vi "Dresden R2R Sputter 03.02.2018 IY24.vi"() -> ()   [LabVIEW 2009] (continued)
        n9883 = Build Array(i32? 49407 ("element")) -> (w15888)
        n9884 = call <vilib>:"MB Serial Master Query Write Multiple Registers (poly).vi"(0:w15891, 1:i16? 320 ("Starting Address"), 2:w15888, 5:w15892, 6:w15880) -> (14:w15882, 19:w15881)  [unwired: 12 in, 1 out]
      }
      frame #9 {
        w15902 = data[3B] ("Serial Parameters")
        n9885 = Type Cast(type=data[3B], x="TC2_overspeed_value") -> (*(type *) &x=w15894)
        n9886 = Build Array(w15894) -> (w15895)
        n9887 = Increment(x=i16? 130) -> (x+1=w15899)
        n9888 = call <vilib>:"MB Serial Master Query Write Multiple Registers (poly).vi"(0:w15901, 1:w15899, 2:w15895, 5:w15900, 6:w15902) -> (14:w15909, 19:w15908)  [unwired: 12 in, 1 out]
        n9889 = local write "TC2_overspeed_set"(i16? 0 ("TC2_overspeed_set")) -> ()
        n9890 = Build Array(i32? 49152 ("element")) -> (w15907)
        n9891 = call <vilib>:"MB Serial Master Query Write Multiple Registers (poly).vi"(0:w15909, 1:i16? 320 ("Starting Address"), 2:w15907, 5:w15908, 6:w15902) -> (14:w15913, 19:w15914)  [unwired: 12 in, 1 out]
        n9892 = Build Array(i32? 49407 ("element")) -> (w15910)
        n9893 = call <vilib>:"MB Serial Master Query Write Multiple Registers (poly).vi"(0:w15913, 1:i16? 320 ("Starting Address"), 2:w15910, 5:w15914, 6:w15902) -> (14:w15904, 19:w15903)  [unwired: 12 in, 1 out]
      }
      frame #10 {
        w15924 = data[3B] ("Serial Parameters")
        n9894 = Type Cast(type=data[3B], x="TC2_AO1_upper_limit_value") -> (*(type *) &x=w15916)
        n9895 = Build Array(w15916) -> (w15917)
        n9896 = Increment(x=i16? 168) -> (x+1=w15921)
        n9897 = call <vilib>:"MB Serial Master Query Write Multiple Registers (poly).vi"(0:w15923, 1:w15921, 2:w15917, 5:w15922, 6:w15924) -> (14:w15931, 19:w15930)  [unwired: 12 in, 1 out]
        n9898 = local write "TC2_AO1_upper_limit_set"(i16? 0 ("TC2_AO1_upper_limit_set")) -> ()
        n9899 = Build Array(i32? 49152 ("element")) -> (w15929)
        n9900 = call <vilib>:"MB Serial Master Query Write Multiple Registers (poly).vi"(0:w15931, 1:i16? 320 ("Starting Address"), 2:w15929, 5:w15930, 6:w15924) -> (14:w15935, 19:w15936)  [unwired: 12 in, 1 out]
        n9901 = Build Array(i32? 49407 ("element")) -> (w15932)
        n9902 = call <vilib>:"MB Serial Master Query Write Multiple Registers (poly).vi"(0:w15935, 1:i16? 320 ("Starting Address"), 2:w15932, 5:w15936, 6:w15924) -> (14:w15926, 19:w15925)  [unwired: 12 in, 1 out]
      }
      frame #11 {
        w15946 = data[3B] ("Serial Parameters")
        n9903 = Type Cast(type=data[3B], x="TC2_AO1_bottom_limit_value") -> (*(type *) &x=w15938)
        n9904 = Build Array(w15938) -> (w15939)
        n9905 = Increment(x=i16? 166) -> (x+1=w15943)
        n9906 = local write "TC2_AO1_bottom_limit_set"(i16? 0 ("TC2_AO1_bottom_limit_set")) -> ()
        n9907 = call <vilib>:"MB Serial Master Query Write Multiple Registers (poly).vi"(0:w15945, 1:w15943, 2:w15939, 5:w15944, 6:w15946) -> (14:w15953, 19:w15952)  [unwired: 12 in, 1 out]
        n9908 = Build Array(i32? 49152 ("element")) -> (w15951)
        n9909 = call <vilib>:"MB Serial Master Query Write Multiple Registers (poly).vi"(0:w15953, 1:i16? 320 ("Starting Address"), 2:w15951, 5:w15952, 6:w15946) -> (14:w15957, 19:w15958)  [unwired: 12 in, 1 out]
        n9910 = Build Array(i32? 49407 ("element")) -> (w15954)
        n9911 = call <vilib>:"MB Serial Master Query Write Multiple Registers (poly).vi"(0:w15957, 1:i16? 320 ("Starting Address"), 2:w15954, 5:w15958, 6:w15946) -> (14:w15948, 19:w15947)  [unwired: 12 in, 1 out]
      }
      frame #12 {
        w15968 = data[3B] ("Serial Parameters")
        n9912 = Type Cast(type=data[3B], x=data[5B] ("TC1_AO1_bottom_limit_value 2")) -> (*(type *) &x=w15960)
        n9913 = Build Array(w15960) -> (w15961)
        n9914 = Increment(x=i16? 198) -> (x+1=w15965)
        n9915 = local write "TC2_AO1_polarity(neg_to_pos)"(i16? 0 ("TC2_AO1_polarity(neg_to_pos)")) -> ()
        n9916 = call <vilib>:"MB Serial Master Query Write Multiple Registers (poly).vi"(0:w15967, 1:w15965, 2:w15961, 5:w15966, 6:w15968) -> (14:w15975, 19:w15974)  [unwired: 12 in, 1 out]
        n9917 = Build Array(i32? 49152 ("element")) -> (w15973)
        n9918 = call <vilib>:"MB Serial Master Query Write Multiple Registers (poly).vi"(0:w15975, 1:i16? 320 ("Starting Address"), 2:w15973, 5:w15974, 6:w15968) -> (14:w15979, 19:w15980)  [unwired: 12 in, 1 out]
        n9919 = Build Array(i32? 49407 ("element")) -> (w15976)
        n9920 = call <vilib>:"MB Serial Master Query Write Multiple Registers (poly).vi"(0:w15979, 1:i16? 320 ("Starting Address"), 2:w15976, 5:w15980, 6:w15968) -> (14:w15970, 19:w15969)  [unwired: 12 in, 1 out]
      }
      frame #13 {
        w15990 = data[3B] ("Serial Parameters")
        n9921 = Type Cast(type=data[3B], x=sgl? 1 ("TC1_AO1_bottom_limit_value 2")) -> (*(type *) &x=w15982)
        n9922 = Build Array(w15982) -> (w15983)
        n9923 = Increment(x=i16? 198) -> (x+1=w15987)
        n9924 = local write "TC2_AO1_polarity(pos_to_neg)"(i16? 0 ("TC2_AO1_polarity(pos_to_neg)")) -> ()
        n9925 = call <vilib>:"MB Serial Master Query Write Multiple Registers (poly).vi"(0:w15989, 1:w15987, 2:w15983, 5:w15988, 6:w15990) -> (14:w15997, 19:w15996)  [unwired: 12 in, 1 out]
        n9926 = Build Array(i32? 49152 ("element")) -> (w15995)
        n9927 = call <vilib>:"MB Serial Master Query Write Multiple Registers (poly).vi"(0:w15997, 1:i16? 320 ("Starting Address"), 2:w15995, 5:w15996, 6:w15990) -> (14:w16001, 19:w16002)  [unwired: 12 in, 1 out]
        n9928 = Build Array(i32? 49407 ("element")) -> (w15998)
        n9929 = call <vilib>:"MB Serial Master Query Write Multiple Registers (poly).vi"(0:w16001, 1:i16? 320 ("Starting Address"), 2:w15998, 5:w16002, 6:w15990) -> (14:w15992, 19:w15991)  [unwired: 12 in, 1 out]
      }
      frame #14 {
        w16012 = data[3B] ("Serial Parameters")
        n9930 = Type Cast(type=data[3B], x=sgl? 2 ("TC1_AO1_bottom_limit_value 2")) -> (*(type *) &x=w16004)
        n9931 = local write "TC2_display_tension_set"(i16? 0 ("TC2_display_tension")) -> ()
        n9932 = Build Array(w16004) -> (w16005)
        n9933 = Increment(x=i16? 8) -> (x+1=w16009)
        n9934 = call <vilib>:"MB Serial Master Query Write Multiple Registers (poly).vi"(0:w16011, 1:w16009, 2:w16005, 5:w16010, 6:w16012) -> (14:w16019, 19:w16018)  [unwired: 12 in, 1 out]
        n9935 = Build Array(i32? 49152 ("element")) -> (w16017)
        n9936 = call <vilib>:"MB Serial Master Query Write Multiple Registers (poly).vi"(0:w16019, 1:i16? 320 ("Starting Address"), 2:w16017, 5:w16018, 6:w16012) -> (14:w16023, 19:w16024)  [unwired: 12 in, 1 out]
        n9937 = Build Array(i32? 49407 ("element")) -> (w16020)
        n9938 = call <vilib>:"MB Serial Master Query Write Multiple Registers (poly).vi"(0:w16023, 1:i16? 320 ("Starting Address"), 2:w16020, 5:w16024, 6:w16012) -> (14:w16014, 19:w16013)  [unwired: 12 in, 1 out]
      }
      frame #15 {
        w16034 = data[3B] ("Serial Parameters")
        n9939 = Type Cast(type=data[3B], x=sgl? 5 ("TC1_AO1_bottom_limit_value 2")) -> (*(type *) &x=w16026)
        n9940 = Build Array(w16026) -> (w16027)
        n9941 = Increment(x=i16? 8) -> (x+1=w16031)
        n9942 = call <vilib>:"MB Serial Master Query Write Multiple Registers (poly).vi"(0:w16033, 1:w16031, 2:w16027, 5:w16032, 6:w16034) -> (14:w16041, 19:w16040)  [unwired: 12 in, 1 out]
        n9943 = local write "TC2_display_AO1_set"(i16? 0 ("TC2_display_tension")) -> ()
        n9944 = Build Array(i32? 49152 ("element")) -> (w16039)
        n9945 = call <vilib>:"MB Serial Master Query Write Multiple Registers (poly).vi"(0:w16041, 1:i16? 320 ("Starting Address"), 2:w16039, 5:w16040, 6:w16034) -> (14:w16045, 19:w16046)  [unwired: 12 in, 1 out]
        n9946 = Build Array(i32? 49407 ("element")) -> (w16042)
        n9947 = call <vilib>:"MB Serial Master Query Write Multiple Registers (poly).vi"(0:w16045, 1:i16? 320 ("Starting Address"), 2:w16042, 5:w16046, 6:w16034) -> (14:w16036, 19:w16035)  [unwired: 12 in, 1 out]
      }
      frame #16 {
        w16056 = data[3B] ("Serial Parameters")
        n9948 = Type Cast(type=data[3B], x=sgl? 4 ("TC1_AO1_bottom_limit_value 2")) -> (*(type *) &x=w16048)
        n9949 = local write "TC2_display_tension_actual"(i16? 0 ("TC2_display_tension")) -> ()
        n9950 = Build Array(w16048) -> (w16049)
        n9951 = Increment(x=i16? 10) -> (x+1=w16053)
        n9952 = call <vilib>:"MB Serial Master Query Write Multiple Registers (poly).vi"(0:w16055, 1:w16053, 2:w16049, 5:w16054, 6:w16056) -> (14:w16063, 19:w16062)  [unwired: 12 in, 1 out]
        n9953 = Build Array(i32? 49152 ("element")) -> (w16061)
        n9954 = call <vilib>:"MB Serial Master Query Write Multiple Registers (poly).vi"(0:w16063, 1:i16? 320 ("Starting Address"), 2:w16061, 5:w16062, 6:w16056) -> (14:w16067, 19:w16068)  [unwired: 12 in, 1 out]
        n9955 = Build Array(i32? 49407 ("element")) -> (w16064)
        n9956 = call <vilib>:"MB Serial Master Query Write Multiple Registers (poly).vi"(0:w16067, 1:i16? 320 ("Starting Address"), 2:w16064, 5:w16068, 6:w16056) -> (14:w16058, 19:w16057)  [unwired: 12 in, 1 out]
      }
      frame #17 {
        w16078 = data[3B] ("Serial Parameters")
        n9957 = Type Cast(type=data[3B], x=data[5B] ("TC1_AO1_bottom_limit_value 2")) -> (*(type *) &x=w16070)
        n9958 = Build Array(w16070) -> (w16071)
        n9959 = Increment(x=i16? 10) -> (x+1=w16075)
        n9960 = call <vilib>:"MB Serial Master Query Write Multiple Registers (poly).vi"(0:w16077, 1:w16075, 2:w16071, 5:w16076, 6:w16078) -> (14:w16085, 19:w16084)  [unwired: 12 in, 1 out]
        n9961 = local write "TC2_display_AO1_actual"(i16? 0 ("TC2_display_tension")) -> ()
        n9962 = Build Array(i32? 49152 ("element")) -> (w16083)
        n9963 = call <vilib>:"MB Serial Master Query Write Multiple Registers (poly).vi"(0:w16085, 1:i16? 320 ("Starting Address"), 2:w16083, 5:w16084, 6:w16078) -> (14:w16089, 19:w16090)  [unwired: 12 in, 1 out]
        n9964 = Build Array(i32? 49407 ("element")) -> (w16086)
        n9965 = call <vilib>:"MB Serial Master Query Write Multiple Registers (poly).vi"(0:w16089, 1:i16? 320 ("Starting Address"), 2:w16086, 5:w16090, 6:w16078) -> (14:w16080, 19:w16079)  [unwired: 12 in, 1 out]
      }
      frame #18 {
        n9966 = Build Array(i16? 21767) -> (w16097)
        n9967 = call <vilib>:"MB Serial Master Query Write Multiple Registers (poly).vi"(0:w16099, 1:i16? 322 ("x"), 2:w16097, 5:w16098, 6:data[3B] ("Serial Parameters")) -> (14:w16092, 19:w16093)  [unwired: 12 in, 1 out]
        n9968 = local write "TC2_tare_function"(i16? 0 ("TC2_tare_function")) -> ()
        n9969 = Build Array(i32? 49407 ("element")) -> (w16102)
        n9970 = call <vilib>:"MB Serial Master Query Write Multiple Registers (poly).vi"(0:w16092, 1:i16? 320 ("Starting Address"), 2:w16102, 5:w16093) -> (14:w16101, 19:w16100)  [unwired: 13 in, 1 out]
      }
    }
  }
  n9971 = while {
    tunnel: [w16539] -> w773
    tunnel: [w16538] -> w745
    tunnel: w772 -> [w16537]
    tunnel: w746 -> [w16536]
    tunnel: "milliseconds to wait 3" -> [w16534]
    stop <- FALSE stop-if-true
    n9972 = stacked-sequence {
      tunnel: [w16544 _] -> w16539
      tunnel: [w16543 _] -> w16538
      tunnel: w16537 -> [w16542 _]
      tunnel: w16536 -> [w16541 _]
      tunnel: w16534 -> [w16540 _]
      frame #0 {
        n9973 = stacked-sequence {
          tunnel: w16541 -> [w16563 _ _ _ _ _ _ _ _ _]
          tunnel: w16542 -> [w16562 _ _ _ _ _ _ _ _ _]
          tunnel: [_ _ _ _ _ _ _ _ w16901 _] -> w16543
          tunnel: [_ _ _ _ _ _ _ _ w16900 _] -> w16544
          tunnel: w16540 -> [_ w16637 _ w16656 _ w16711 _ w16887 _ w16920]
          frame #0 {
            # "Digital I/O & Analog \nOutput Part"
            n9974 = call-poly <vilib>:"MB Serial Master Query (poly).vi"("VISA resource name"=w16563, "Starting Address"=u16 0, "Quantity"=u16 8, "error in"=w16562, "Serial Parameters"=T39 {"Mode"=enum."RTU", "Slave Address"=1}) -> ("VISA resource name out"=w16560:refnum<visa-resource-name>, "Discrete Inputs"=w16590:bool[], "error out"=w16561:errorcluster)  [unwired: 1 in, 11 out]
            n9975 = Index Array(array=w16590, index=5) -> (element=w16553:bool)
            "Ch2_Pl_vbv_di" <- w16553
            n9976 = Index Array(array=w16590, index=6) -> (element=w16585:bool)
            "Ch2_Pl_atm_di" <- w16585
            n9977 = Index Array(array=w16590, index=0) -> (element=w16588:bool)
            "Ch2_Mp_di" <- w16588
            n9978 = Index Array(array=w16590, index=1) -> (element=w16587:bool)
            "Ch2_Tp_bv_di" <- w16587
            n9979 = Index Array(array=w16590, index=2) -> (element=w16550:bool)
            "Ch2_Bg_bv_di" <- w16550
            n9980 = Index Array(array=w16590, index=3) -> (element=w16586:bool)
            "Ch2_Ch_vbv_di" <- w16586
            n9981 = Index Array(array=w16590, index=4) -> (element=w16549:bool)
            "Ch2_Ch_atm_di" <- w16549
            n9982 = Index Array(array=w16590, index=7) -> (element=w16548:bool)
            "Ch2_Cc_on_off_di" <- w16548
            n9983 = local write "Ch2_Ch_vbv_on"(w16586) -> ()
            n9984 = local write "Ch2_Ch_atm_on"(w16549) -> ()
            n9985 = local write "Ch2_Bg_bv_on"(w16550) -> ()
            n9986 = local write "ch2_bg_bv_on_top"(w16550) -> ()
            n9987 = local write "ch2_cc_on_top"(w16548) -> ()
            n9988 = local write "Ch2_Tp_bv_on"(w16587) -> ()
            n9989 = local write "Ch2_Pl_atm_on"(w16585) -> ()
            n9990 = local write "Ch2_Ch_cc_on"(w16548) -> ()
            n9991 = local write "Ch2_Mp_on"(w16588) -> ()
            n9992 = local write "Ch2_Pl_vbv_on"(w16553) -> ()
            n9993 = local write "ch2_atm_on_top"(w16549) -> ()
            n9994 = local read "Load_dido"() -> (w16552:bool)
            n9995 = call-poly <vilib>:"MB Serial Master Query (poly).vi"("VISA resource name"=w16560, "Starting Address"=u16 0, "Quantity"=u16 8, "error in"=w16561, "Serial Parameters"=T39 {"Mode"=enum."RTU", "Slave Address"=2}) -> ("VISA resource name out"=w16558:refnum<visa-resource-name>, "Discrete Inputs"=w16607:bool[], "error out"=w16559:errorcluster)  [unwired: 1 in, 11 out]
            n9996 = case shown="True" w16552 {
              frame #0 {
              }
              frame #1 {
                n9997 = Wait (ms)(milliseconds to wait=u32 2000) -> ()  [unwired: 1 out]
              }
            }
            n9998 = Index Array(array=w16607, index=3) -> (element=w16547:bool)
            "Ch2_trns_gv_bp_di" <- w16547
            n9999 = Index Array(array=w16607, index=5) -> (element=w16601:bool)
            "Ch2_Cst_fix_down_di" <- w16601
            n10000 = Index Array(array=w16607, index=0) -> (element=w16551:bool)
            "Ch2_Sov_Ar_di" <- w16551
            n10001 = Index Array(array=w16607, index=1) -> (element=w16545:bool)
            "Ch2_Trns_gv_open_di" <- w16545
            n10002 = Index Array(array=w16607, index=2) -> (element=→"Ch2_Trns_gv_close_di":bool)
            n10003 = Index Array(array=w16607, index=6) -> (element=→"Ch2_Pet_cool_up_di":bool)
            n10004 = Index Array(array=w16607, index=7) -> (element=→"Ch2_Pet_cool_down_di":bool)
            n10005 = Index Array(array=w16607, index=4) -> (element=→"Ch2_Cst_fix_up_di":bool)
            n10006 = local write "gv front open_ch3_2"(w16545) -> ()
            n10007 = local write "gv front open_ch2_3"(w16545) -> ()
            n10008 = local write "gv top on_ch2_3"(w16545) -> ()
            n10009 = local write "Trns_gv_2_3_on"(w16545) -> ()
            n10010 = local write "ch2_sov_Ar_on_top"(w16551) -> ()
            n10011 = local write "gv top_open_ch3_2"(w16545) -> ()
            n10012 = local write "Ch2_trns_gv_bp_on_top"(w16547) -> ()
            n10013 = local write "Ch2_Trns_gv_bp_on"(w16547) -> ()
            n10014 = local write "ch2_trns_gv_bp_on_front"(w16547) -> ()
            n10015 = local write "Ch2_Cst_fix_down"(w16601) -> ()
            n10016 = call-poly <vilib>:"MB Serial Master Query (poly).vi"("VISA resource name"=w16558, "Starting Address"=u16 0, "Quantity"=u16 8, "error in"=w16559, "Serial Parameters"=T39 {"Mode"=enum."RTU", "Slave Address"=3}) -> ("VISA resource name out"=w16556:refnum<visa-resource-name>, "Discrete Inputs"=w16620:bool[], "error out"=w16557:errorcluster)  [unwired: 1 in, 11 out]
            n10017 = Index Array(array=w16620, index=5) -> (element=→"Ch2_SRV2_counter_di":bool)
            n10018 = Index Array(array=w16620, index=6) -> (element=→"Ch2_WFS_di":bool)
            n10019 = Index Array(array=w16620, index=7) -> (element=w16546:bool)
            "Ch2_trns_gv_bp2_di" <- w16546
            n10020 = Index Array(array=w16620, index=0) -> (element=→"Ch2_SRV1_PIST For_di":bool)
            n10021 = Index Array(array=w16620, index=1) -> (element=→"Ch2_SRV1_PIST_Back_di":bool)
            n10022 = Index Array(array=w16620, index=2) -> (element=→"Ch2_SRV_start_stop_di":bool)
            n10023 = Index Array(array=w16620, index=3) -> (element=→"Ch2_SRV_leftdirection(CCW)_di":bool)
            n10024 = Index Array(array=w16620, index=4) -> (element=→"Ch2_SRV1_counter_di":bool)
            n10025 = local write "Ch2_Trns_gv_bp2_on"(w16546) -> ()
            n10026 = local write "Ch2_trns_gv_bp2_top"(w16546) -> ()
            n10027 = local write "ch2_trns_gv_bp2_on_front"(w16546) -> ()
            n10028 = call-poly <vilib>:"MB Serial Master Query (poly).vi"("VISA resource name"=w16556, "Starting Address"=u16 0, "Quantity"=u16 8, "error in"=w16557, "Serial Parameters"=T39 {"Mode"=enum."RTU", "Slave Address"=4}) -> ("VISA resource name out"=w16555:refnum<visa-resource-name>, "Discrete Inputs"=w16571:bool[], "error out"=w16554:errorcluster)  [unwired: 1 in, 11 out]
            n10029 = Index Array(array=w16571, index=5) -> (element=→"Ch2_Right_slow_di":bool)
            n10030 = Index Array(array=w16571, index=6) -> (element=→"Ch2_Left_slow_di":bool)
            n10031 = Index Array(array=w16571, index=7) -> (element=→"Ch2_Left_limit_di":bool)
            n10032 = Index Array(array=w16571, index=0) -> (element=→"Ch2_Air_press_di":bool)
            n10033 = Index Array(array=w16571, index=1) -> (element=→"Ch2_Ds_di":bool)
            n10034 = Index Array(array=w16571, index=2) -> (element=→"Ch2_TGV_control_di":bool)
            n10035 = Index Array(array=w16571, index=3) -> (element=→"Ch2_Trns_interlock_di":bool)
            n10036 = Index Array(array=w16571, index=4) -> (element=→"Ch2_Right_limit_di":bool)
          }
          frame #1 {
            n10037 = Wait (ms)(milliseconds to wait=w16637) -> ()  [unwired: 1 out]
          }
          frame #2 {
            n10038 = local read "Load_dido"() -> (w16638:bool)
            n10039 = case shown="True" w16638 {
              frame #0 {
              }
              frame #1 {
                n10040 = while {
                  stop <- w16648 stop-if-true
                  n10041 = local read "Ch2_Mp_di"() -> (w16655:bool)
                  n10042 = local read "Ch2_Tp_bv_di"() -> (w16654:bool)
                  n10043 = local read "Ch2_Bg_bv_di"() -> (w16653:bool)
                  n10044 = local read "Ch2_Ch_vbv_di"() -> (w16652:bool)
                  n10045 = local read "Ch2_Pl_vbv_di"() -> (w16651:bool)
                  n10046 = local read "Ch2_Cc_on_off_di"() -> (w16650:bool)
                  n10047 = Wait Until Next ms Multiple(millisecond multiple=u32 300) -> ()  [unwired: 1 out]
                  n10048 = local write "Ch2_Mp_do"(w16655) -> ()
                  n10049 = local write "Ch2_Tp_bv_do"(w16654) -> ()
                  n10050 = local write "Ch2_Bg_bv_do"(w16653) -> ()
                  n10051 = local write "Ch2_Ch_vbv_do"(w16652) -> ()
                  n10052 = local write "Ch2_Pl_vbv_do"(w16651) -> ()
                  n10053 = local write "Ch2_Cc_on_off_do"(w16650) -> ()
                  n10054 = local read "Ch2_WFS_di"() -> (w16639:bool)
                  n10055 = local read "Ch2_Sov_Ar_di"() -> (w16640:bool)
                  n10056 = local read "Ch2_Trns_gv_open_di"() -> (w16641:bool)
                  n10057 = local read "Ch2_Trns_gv_close_di"() -> (w16642:bool)
                  n10058 = local read "Ch2_trns_gv_bp_di"() -> (w16646:bool)
                  n10059 = local read "Ch2_Cst_fix_down_di"() -> (w16643:bool)
                  n10060 = local read "Ch2_Pet_cool_up_di"() -> (w16644:bool)
                  n10061 = local read "Ch2_Pet_cool_down_di"() -> (w16645:bool)
                  n10062 = local write "Ch2_WFC_do"(w16639) -> ()
                  n10063 = local write "Ch2_Sov_Ar_do"(w16640) -> ()
                  n10064 = local write "Ch2_Trns_gv_open_do"(w16641) -> ()
                  n10065 = local write "Ch2_Trns_gv_close_do"(w16642) -> ()
                  n10066 = local write "Ch2_Cst_fix_do"(w16643) -> ()
                  n10067 = local write "Ch2_Pet_cool_up_do"(w16644) -> ()
                  n10068 = local write "Ch2_Pet_cool_down_do"(w16645) -> ()
                  n10069 = local write "Ch2_trns_gv_bp_do"(w16646) -> ()
                  n10070 = local read "Load_dido"() -> (w16647:bool)
                  n10071 = Not(x=w16647) -> (.not. x?=w16648:bool)
                }
              }
            }
          }
          frame #3 {
            n10072 = Wait (ms)(milliseconds to wait=w16656) -> ()  [unwired: 1 out]
          }
          frame #4 {
            n10073 = Build Array("Ch2_Mp_do", "Ch2_Tp_bv_do", "Ch2_Bg_bv_do", "Ch2_Ch_vbv_do", "Ch2_Ch_atm_do", "Ch2_Pl_vbv_do", "Ch2_Pl_atm_do", "Ch2_Cc_on_off_do") -> (w16683:bool[])
            n10074 = call-poly <vilib>:"MB Serial Master Query (poly).vi"("VISA resource name"=w16673, "Starting Address"=u16 320, "Coils"=w16683, "error in"=w16672, "Serial Parameters"=T39 {"Mode"=enum."RTU", "Slave Address"=1}) -> ("VISA resource name out"=w16670:refnum<visa-resource-name>, "error out"=w16669:errorcluster)  [unwired: 1 in, 12 out]
            n10075 = Build Array("Ch2_Sov_Ar_do", "Ch2_Trns_gv_open_do", "Ch2_Trns_gv_close_do", "Ch2_trns_gv_bp_do", "Ch2_Cst_fix_do", "Ch2_2_5_do", "Ch2_Pet_cool_up_do", "Ch2_Pet_cool_down_do") -> (w16684:bool[])
            n10076 = call-poly <vilib>:"MB Serial Master Query (poly).vi"("VISA resource name"=w16670, "Starting Address"=u16 320, "Coils"=w16684, "error in"=w16669, "Serial Parameters"=T39 {"Mode"=enum."RTU", "Slave Address"=2}) -> ("VISA resource name out"=w16667:refnum<visa-resource-name>, "error out"=w16668:errorcluster)  [unwired: 1 in, 12 out]
            n10077 = Build Array("Ch2_SRV1_PIST For_do", "Ch2_SRV1_PIST_Back_do", "Ch2_SRV_start_stop_do", "Ch2_SRV_counterclockwise_direction_do", "Ch2_3_4_do", "Ch2_3_5_do", "Ch2_WFC_do", "Ch2_trns_gv_bp2_do") -> (w16702:bool[])
            n10078 = call-poly <vilib>:"MB Serial Master Query (poly).vi"("VISA resource name"=w16667, "Starting Address"=u16 320, "Coils"=w16702, "error in"=w16668, "Serial Parameters"=T39 {"Mode"=enum."RTU", "Slave Address"=3}) -> ("VISA resource name out"=w16665:refnum<visa-resource-name>, "error out"=w16664:errorcluster)  [unwired: 1 in, 12 out]
            n10079 = Build Array("Ch2_4_0_do", "Ch2_4_1_do", "Ch2_TGV_control_do", "Ch2_4_3_do", "Ch2_4_4_do", "Ch2_4_5_do", "Ch2_4_6_do", "Ch2_4_7_do") -> (w16703:bool[])
            n10080 = call-poly <vilib>:"MB Serial Master Query (poly).vi"("VISA resource name"=w16665, "Starting Address"=u16 320, "Coils"=w16703, "error in"=w16664, "Serial Parameters"=T39 {"Mode"=enum."RTU", "Slave Address"=4}) -> ("VISA resource name out"=w16662:refnum<visa-resource-name>, "error out"=w16661:errorcluster)  [unwired: 1 in, 12 out]
          }
          frame #5 {
            n10081 = Wait (ms)(milliseconds to wait=w16711) -> ()  [unwired: 1 out]
          }
          frame #6 {
            n10082 = call-poly <vilib>:"MB Serial Master Query (poly).vi"("VISA resource name"=w16720, "Starting Address"=u16 704, "Quantity"=u16 8, "error in"=w16718, "Serial Parameters"=T39 {"Mode"=enum."RTU", "Slave Address"=5}) -> ("VISA resource name out"=w16719:refnum<visa-resource-name>, "Input Registers"=w16732:u16[], "error out"=w16717:errorcluster)  [unwired: 1 in, 11 out]
            n10083 = local read "1bit="() -> (w16714:dbl)
            n10084 = local read "1bit="() -> (w16722:dbl)
            n10085 = Index Array(array=w16732, index=5) -> (element=→"Ch1_Ai_1_5 2":u16)
            n10086 = Index Array(array=w16732, index=6) -> (element=→"Ch1_Ai_1_6 2":u16)
            n10087 = Index Array(array=w16732, index=7) -> (element=→"Ch1_Ai_1_7 2":u16)
            n10088 = Index Array(array=w16732, index=0) -> (element=w16727:u16)
            "Ch2_Ai_PL_PG" <- w16727
            n10089 = Index Array(array=w16732, index=1) -> (element=w16715:u16)
            "Ch2_Ai_CH_PG" <- w16715
            n10090 = Index Array(array=w16732, index=2) -> (element=w16716:u16)
            "Ch2_Ai_CH-CC" <- w16716
            n10091 = Index Array(array=w16732, index=3) -> (element=w16713:u16)
            "Ch2_Ai_MFC_Ar_2" <- w16713
            n10092 = Multiply(x=w16714, y=w16713) -> (x*y=w16712:dbl)
            n10093 = Index Array(array=w16732, index=4) -> (element=→"Ch1_Ai_1_4 2":u16)
            n10094 = Multiply(x=w16722, y=w16716) -> (x*y=w16721:dbl)
            n10095 = stacked-sequence {
              tunnel: w16721 -> [w16771]
              frame #0 {
                # "CH-CC 0-10 Volt okuma"
                n10096 = feedback #351() -> (w16780:dbl)  [unwired: 1 in]
                n10097 = feedback #352() -> (w16781:dbl)  [unwired: 1 in]
                n10098 = feedback #353() -> (w16782:dbl)  [unwired: 1 in]
                n10099 = feedback #354() -> (w16783:dbl)  [unwired: 1 in]
                n10100 = feedback #355() -> (w16784:dbl)  [unwired: 1 in]
                n10101 = feedback #356() -> (w16785:dbl)  [unwired: 1 in]
                n10102 = feedback #357() -> (w16769:dbl)  [unwired: 1 in]
                n10103 = feedback #358() -> (w16796:dbl)  [unwired: 1 in]
                n10104 = feedback #359() -> (w16786:dbl)  [unwired: 1 in]
                n10105 = feedback #360() -> (w16787:dbl)  [unwired: 1 in]
                n10106 = feedback #361() -> (w16788:dbl)  [unwired: 1 in]
                n10107 = feedback #362() -> (w16789:dbl)  [unwired: 1 in]
                n10108 = feedback #363() -> (w16790:dbl)  [unwired: 1 in]
                n10109 = feedback #364() -> (w16791:dbl)  [unwired: 1 in]
                n10110 = feedback #365() -> (w16792:dbl)  [unwired: 1 in]
                n10111 = feedback #366() -> (w16770:dbl)  [unwired: 1 in]
                n10112 = feedback #367() -> (w16793:dbl)  [unwired: 1 in]
                n10113 = feedback #368() -> (w16794:dbl)  [unwired: 1 in]
                n10114 = feedback #369() -> (w16795:dbl)  [unwired: 1 in]
                n10115 = Compound Arithmetic op=ADD(w16771, w16780, w16781, w16782, w16783, w16784, w16785, w16769, w16796, w16786, w16787, w16788, w16789, w16790, w16791, w16792, w16770, w16793, w16794, w16795) -> (w16779:dbl)
                n10116 = Divide(x=w16779, y=u16 20) -> (x/y=w16775:dbl)
                "Ch_CC_volt ch2" <- w16775
                n10117 = feedback #370() -> (w16772:bool)  [unwired: 1 in]
                n10118 = Greater?(x=w16775, y=1.0) -> (0:w16776:bool)
                n10119 = case shown="True" w16776 {
                  tunnel: w16775 -> [_ w16813]
                  tunnel: [w16804 FALSE] -> w16774
                  tunnel: [FALSE ("Ch_cc_on(ch1)") TRUE] -> w16773
                  tunnel: w16772 -> [_ _]
                  frame #0 {
                    n10120 = local read "Ch2_Cc_on_off_di"() -> (w16798:bool)
                    n10121 = call "Elapsed Time90"() -> ("Elapsed Time (s)"=w16807:dbl)  [unwired: 12 in, 7 out]
                    n10122 = local write "Ch2_Ch_cc_on"(FALSE ("Ch_cc_on(ch1)")) -> ()
                    n10123 = Not(x=w16798) -> (.not. x?=w16801:bool)
                    n10124 = Greater Or Equal?(x=w16807, y=3.0) -> (x >= y?=w16806:bool)
                    n10125 = call "Elapsed Time91"("Reset"=w16801) -> ("Elapsed Time (s)"=w16803:dbl)  [unwired: 11 in, 7 out]
                    n10126 = Greater Or Equal?(x=w16803, y=3.0) -> (x >= y?=w16800:bool)
                    n10127 = And(x=w16806, y=w16800) -> (x .and. y?=w16804:bool)
                  }
                  frame #1 {
                    (unwired) 10.0 ("x")
                    n10128 = Subtract(x=w16813, y=10.625) -> (x-y=w16810:dbl)
                    n10129 = Power Of 10(x=w16810) -> (10^x=w16809:dbl)
                    n10130 = In Range and Coerce(upper limit=0.0075, x=w16809, lower limit=1.5e-09) -> (coerced(x)=→"Ch_CC_press_ch2" →"Ch_CC_press_ch2 2":dbl)  [unwired: 1 out]
                  }
                }
                n10131 = local write "Ch2_Ch_cc_fail"(w16774) -> ()
                "Ch_CC_volt_intantaneous_ch2" <- w16771
              }
            }
            n10132 = local read "1bit="() -> (w16726:dbl)
            n10133 = local read "1bit="() -> (w16724:dbl)
            n10134 = stacked-sequence {
              tunnel: w16712 -> [w16745]
              frame #0 {
                # "MFC AR 0-5 volt okuma"
                n10135 = feedback #371() -> (w16750:dbl)  [unwired: 1 in]
                n10136 = feedback #372() -> (w16751:dbl)  [unwired: 1 in]
                n10137 = feedback #373() -> (w16752:dbl)  [unwired: 1 in]
                n10138 = feedback #374() -> (w16753:dbl)  [unwired: 1 in]
                n10139 = Compound Arithmetic op=ADD(w16745, w16750, w16751, w16752, w16753) -> (w16749:dbl)
                n10140 = Divide(x=w16749, y=u16 5) -> (x/y=w16744:dbl)
                "MFC_volt" <- w16744
                n10141 = Greater?(x=w16744, y=0.1) -> (0:w16746:bool)
                n10142 = case shown="False" w16746 {
                  tunnel: w16744 -> [_ w16757]
                  frame #0 {
                    w16754 = 0.0 ("Ar_sccm_act")
                    n10143 = local write "Ar_sccm_act gui"(w16754) -> ()
                    n10144 = local write "Ar_sccm_act 6"(w16754) -> ()
                    n10145 = local write "Ar_sccm_act 5"(w16754) -> ()
                  }
                  frame #1 {
                    # "200 ccm/5V\nçarpan 40"
                    n10146 = Multiply(x=w16757, y=40.0) -> (x*y=→"Ar_sccm_act 6" →"Ar_sccm_act gui" →"Ar_sccm_act 5":dbl)
                  }
                }
                "MFC_volt_instantaneous" <- w16745
              }
            }
            n10147 = Multiply(x=w16726, y=w16727) -> (x*y=w16725:dbl)
            n10148 = Multiply(x=w16724, y=w16715) -> (x*y=w16723:dbl)
            n10149 = stacked-sequence {
              tunnel: w16723 -> [w16824]
              frame #0 {
                # "CH-PG 0-10 Volt okuma"
                n10150 = feedback #375() -> (w16835:dbl)  [unwired: 1 in]
                n10151 = feedback #376() -> (w16833:dbl)  [unwired: 1 in]
                n10152 = feedback #377() -> (w16832:dbl)  [unwired: 1 in]
                n10153 = feedback #378() -> (w16831:dbl)  [unwired: 1 in]
                n10154 = feedback #379() -> (w16830:dbl)  [unwired: 1 in]
                n10155 = feedback #380() -> (w16829:dbl)  [unwired: 1 in]
                n10156 = feedback #381() -> (w16828:dbl)  [unwired: 1 in]
                n10157 = feedback #382() -> (w16826:dbl)  [unwired: 1 in]
                n10158 = feedback #383() -> (w16827:dbl)  [unwired: 1 in]
                n10159 = Compound Arithmetic op=ADD(w16824, w16835, w16833, w16832, w16831, w16830, w16829, w16828, w16826, w16827) -> (w16834:dbl)
                n10160 = Divide(x=w16834, y=u16 10) -> (x/y=w16818:dbl)
                "Ch_pg_volt_ch2" <- w16818
                n10161 = local read "Ch_pg_volt_intantaneous_ch2"() -> (w16817:u16)
                n10162 = Greater Or Equal?(x=w16817, y=u16 1) -> (x >= y?=w16819:bool)
                n10163 = feedback #384() -> (w16822:bool)  [unwired: 1 in]
                n10164 = case shown="True" w16819 {
                  tunnel: w16818 -> [_ w16847]
                  tunnel: [FALSE TRUE] -> w16821
                  tunnel: w16822 -> [w16838 _]
                  tunnel: [w16837 FALSE ("Bg_gui")] -> w16823
                  frame #0 {
                    n10165 = call "Elapsed Time141"("Reset"=w16838) -> ("Elapsed Time (s)"=w16841:dbl)  [unwired: 11 in, 7 out]
                    n10166 = local write "Ch2_Ch_pg_on"(FALSE ("Bg_gui")) -> ()
                    n10167 = Greater Or Equal?(x=w16841, y=3.0) -> (x >= y?=w16837:bool)
                  }
                  frame #1 {
                    n10168 = Subtract(x=w16847, y=5.625) -> (x-y=w16849:dbl)
                    n10169 = Power Of 10(x=w16849) -> (10^x=w16848:dbl)
                    n10170 = In Range and Coerce(upper limit=760.0, x=w16848, lower limit=0.000375) -> (coerced(x)=→"Ch_pg_press_ch2" →"Ch_pg_press_ch2_gui" →"Ch_pg_press_ch2_gui 2":dbl)  [unwired: 1 out]
                    n10171 = local write "Ch2_Ch_pg_on"(TRUE ("Bg_gui")) -> ()
                  }
                }
                n10172 = local write "Ch2_Ch_pg_fail"(w16823) -> ()
                "Ch_pg_volt_intantaneous_ch2" <- w16824
              }
            }
            n10173 = stacked-sequence {
              tunnel: w16725 -> [w16860]
              frame #0 {
                # "PL-PG 0-10 Volt okuma"
                n10174 = feedback #385() -> (w16870:dbl)  [unwired: 1 in]
                n10175 = feedback #386() -> (w16868:dbl)  [unwired: 1 in]
                n10176 = feedback #387() -> (w16867:dbl)  [unwired: 1 in]
                n10177 = feedback #388() -> (w16866:dbl)  [unwired: 1 in]
                n10178 = feedback #389() -> (w16865:dbl)  [unwired: 1 in]
                n10179 = feedback #390() -> (w16864:dbl)  [unwired: 1 in]
                n10180 = feedback #391() -> (w16863:dbl)  [unwired: 1 in]
                n10181 = feedback #392() -> (w16862:dbl)  [unwired: 1 in]
                n10182 = feedback #393() -> (w16852:dbl)  [unwired: 1 in]
                n10183 = Compound Arithmetic op=ADD(w16860, w16870, w16868, w16867, w16866, w16865, w16864, w16863, w16862, w16852) -> (w16869:dbl)
                n10184 = local read "Pl_pg_volt_instantaneous_ch2"() -> (w16858:u16)
                n10185 = Divide(x=w16869, y=10.0) -> (x/y=w16859:dbl)
                "Pl_pg_volt_ch2" <- w16859
                n10186 = Greater Or Equal?(x=w16858, y=u16 1) -> (x >= y?=w16857:bool)
                n10187 = feedback #394() -> (w16854:bool)  [unwired: 1 in]
                n10188 = case shown="True" w16857 {
                  tunnel: w16859 -> [_ w16882]
                  tunnel: [FALSE TRUE] -> w16855
                  tunnel: w16854 -> [w16873 _]
                  tunnel: [w16872 FALSE ("Bg_gui")] -> w16853
                  frame #0 {
                    n10189 = call "Elapsed Time86"("Reset"=w16873) -> ("Elapsed Time (s)"=w16876:dbl)  [unwired: 11 in, 7 out]
                    n10190 = local write "Ch2_Pl_pg_on"(FALSE ("Bg_gui")) -> ()
                    n10191 = Greater Or Equal?(x=w16876, y=3.0) -> (x >= y?=w16872:bool)
                  }
                  frame #1 {
                    n10192 = Subtract(x=w16882, y=5.625) -> (x-y=w16884:dbl)
                    n10193 = Power Of 10(x=w16884) -> (10^x=w16883:dbl)
                    n10194 = In Range and Coerce(upper limit=760.0, x=w16883, lower limit=0.000375) -> (coerced(x)=→"Pl_pg_press_ch2" →"Pl_pg_press_ch2_gui":dbl)  [unwired: 1 out]
                    n10195 = local write "Ch2_Pl_pg_on"(TRUE ("Bg_gui")) -> ()
                  }
                }
                n10196 = local write "Ch2_Pl_pg_fail"(w16853) -> ()
                "Pl_pg_volt_instantaneous_ch2" <- w16860
              }
            }
            n10197 = stacked-sequence {
              frame #0 {
                n10198 = local read "Ch2_Cc_on_off_di"() -> (w16758:bool)
                n10199 = case shown="True" w16758 {
                  frame #0 {
                    n10200 = local read "Ch_pg_press_ch2"() -> (→"Ch2_pressure" →"Ch2_pressure2":dbl)
                  }
                  frame #1 {
                    n10201 = local read "Ch_CC_volt ch2"() -> (w16766:u16)
                    n10202 = local read "Ch_pg_volt_ch2"() -> (w16765:u16)
                    n10203 = Greater?(x=w16766, y=1.8) -> (0:w16764:bool)
                    n10204 = Less?(x=w16765, y=u16 2) -> (x < y?=w16763:bool)
                    n10205 = Or(x=w16764, y=w16763) -> (x .or. y?=w16762:bool)
                    n10206 = case shown="True" w16762 {
                      frame #0 {
                        n10207 = local read "Ch_pg_press_ch2"() -> (w16767:dbl)
                        n10208 = local write "Ch2_pressure2"(w16767) -> ()
                        n10209 = local write "Ch2_pressure"(w16767) -> ()
                      }
                      frame #1 {
                        n10210 = local read "Ch_CC_press_ch2"() -> (w16768:dbl)
                        n10211 = local write "Ch2_pressure"(w16768) -> ()
                        n10212 = local write "Ch2_pressure2"(w16768) -> ()
                      }
                    }
                  }
                }
              }
            }
          }
          frame #7 {
            n10213 = Wait (ms)(milliseconds to wait=w16887) -> ()  [unwired: 1 out]
          }
          frame #8 {
            n10214 = Build Array(FALSE, "Ch2_Ao_1_0", "Ch2_Ao_1_1", "Ch2_Ao_1_2", "Mfc_Ar _1_2_set") -> (w16894:bool[])
            n10215 = Boolean Array To Number(Boolean array=w16894) -> (number=w16899:u32)
            n10216 = Mantissa & Exponent(0:w16899) -> (2:w16893:dbl)  [unwired: 1 out]
            n10217 = case shown="4" w16893 {
              tunnel: [u16 0 ("Starting Address") u16 1184 ("Starting Address") u16 1185 ("Starting Address") u16 1186 ("Starting Address") u16 1187 ("Starting Address")] -> w16902
              tunnel: [u16 0 ("Ao_1_3") "Ch2_Ao_1_0 2" "Ch2_Ao_1_1 2" "Ch2_Ao_1_2 2" w16912] -> w16892
              frame #0 {
              }
              frame #1 {
              }
              frame #2 {
              }
              frame #3 {
              }
              frame #4 {
                n10218 = Divide(x=2048.0, y=200.0) -> (x/y=w16916:dbl)
                n10219 = flat-sequence {
                  frame #0 {
                    n10220 = Wait (ms)(milliseconds to wait=u32 100) -> ()  [unwired: 1 out]
                  }
                  frame #1 {
                    n10221 = local write "Mfc_Ar _1_2_set"(FALSE ("Mfc_Ar _set")) -> ()
                  }
                }
                n10222 = Multiply(x="Ar_sccm1_2", y=w16916) -> (x*y=w16912:dbl)
              }
            }
            n10223 = Build Array(w16892) -> (w16891:dbl[])
            n10224 = call-poly <vilib>:"MB Serial Master Query (poly).vi"("VISA resource name"=w16890, "Starting Address"=w16902, "Registers"=w16891, "error in"=w16889, "Serial Parameters"=T39 {"Mode"=enum."RTU", "Slave Address"=6}) -> ("VISA resource name out"=w16901:refnum<visa-resource-name>, "error out"=w16900:errorcluster)  [unwired: 1 in, 12 out]
          }
          frame #9 {
            n10225 = Wait (ms)(milliseconds to wait=w16920) -> ()  [unwired: 1 out]
          }
        }
      }
      frame #1 {
        n10226 = local read "Fail_moxa2_digital2"() -> (w16924:bool)
        n10227 = local read "Fail_moxa2_digital3"() -> (w16923:bool)
        n10228 = local read "Fail_moxa2_digital4"() -> (w16922:bool)
        n10229 = local read "Fail_moxa2_digital1"() -> (w16921:bool)
        n10230 = case shown="False" w16924 {
          frame #0 {
            w16940 = TRUE
            n10231 = local write "Ch2_trns_gv_bp_fail_top"(w16940) -> ()
            n10232 = local write "ch2_sov_Ar_fail_top"(w16940) -> ()
            n10233 = local write "Trns_gv_2_3_fail"(w16940) -> ()
            n10234 = local write "ch2_trns_gv_bp_fail_front"(w16940) -> ()
            n10235 = local write "gv top failed_ch3_2"(w16940) -> ()
            n10236 = local write "gv front failed_ch3_2"(w16940) -> ()
            n10237 = local write "gv front failed_ch2_3"(w16940) -> ()
            n10238 = local write "gv top failed_ch2_3"(w16940) -> ()
            n10239 = local write "Ch2_Trns_gv_bp_fail"(w16940) -> ()
            n10240 = local write "chamber 2top piston failed"(w16940) -> ()
          }
          frame #1 {
            n10241 = local read "Ch2_Sov_Ar_do"() -> (w16960:bool)
            n10242 = local read "Ch2_Sov_Ar_di"() -> (w16961:bool)
            n10243 = Exclusive Or(1:w16960, 2:w16961) -> (0:w16962:bool)
            n10244 = feedback #395() -> (w16963:bool)  [unwired: 1 in]
            n10245 = case shown="True" w16962 {
              tunnel: [TRUE FALSE] -> w16964
              tunnel: w16963 -> [_ w16991]
              tunnel: [FALSE w16988] -> w16947
              frame #0 {
              }
              frame #1 {
                n10246 = call "Elapsed Time112"("Reset"=w16991) -> ("Elapsed Time (s)"=w16990:dbl)  [unwired: 11 in, 7 out]
                n10247 = Greater?(x=w16990, y=5.0) -> (0:w16988:bool)
              }
            }
            n10248 = local write "ch2_sov_Ar_fail_top"(w16947) -> ()
            n10249 = local read "Ch2_Trns_gv_open_di"() -> (w16958:bool)
            n10250 = local read "Ch2_Trns_gv_open_do"() -> (w16959:bool)
            n10251 = Exclusive Or(1:w16959, 2:w16958) -> (0:w16957:bool)
            n10252 = feedback #396() -> (w16956:bool)  [unwired: 1 in]
            n10253 = case shown="True" w16957 {
              tunnel: [TRUE FALSE] -> w16955
              tunnel: w16956 -> [_ w16984]
              tunnel: [FALSE w16981] -> w16954
              frame #0 {
              }
              frame #1 {
                n10254 = call "Elapsed Time136"("Reset"=w16984) -> ("Elapsed Time (s)"=w16983:dbl)  [unwired: 11 in, 7 out]
                n10255 = Greater?(x=w16983, y=60.0) -> (0:w16981:bool)
              }
            }
            n10256 = local write "gv front failed_ch3_2"(w16954) -> ()
            n10257 = local write "gv front failed_ch2_3"(w16954) -> ()
            n10258 = local write "gv top failed_ch2_3"(w16954) -> ()
            n10259 = local write "gv top failed_ch3_2"(w16954) -> ()
            n10260 = local write "Trns_gv_2_3_fail"(w16954) -> ()
            n10261 = local read "Ch2_trns_gv_bp_do"() -> (w16949:bool)
            n10262 = local read "Ch2_trns_gv_bp_di"() -> (w16950:bool)
            n10263 = Exclusive Or(1:w16949, 2:w16950) -> (0:w16951:bool)
            n10264 = feedback #397() -> (w16952:bool)  [unwired: 1 in]
            n10265 = case shown="True" w16951 {
              tunnel: [TRUE FALSE] -> w16953
              tunnel: w16952 -> [_ w16977]
              tunnel: [FALSE w16974] -> w16948
              frame #0 {
              }
              frame #1 {
                n10266 = call "Elapsed Time185"("Reset"=w16977) -> ("Elapsed Time (s)"=w16976:dbl)  [unwired: 11 in, 7 out]
                n10267 = Greater?(x=w16976, y=5.0) -> (0:w16974:bool)
              }
            }
            n10268 = local write "Ch2_Trns_gv_bp_fail"(w16948) -> ()
            n10269 = local write "ch2_trns_gv_bp_fail_front"(w16948) -> ()
            n10270 = local write "Ch2_trns_gv_bp_fail_top"(w16948) -> ()
            n10271 = local read "Ch2_Cst_fix_down_di"() -> (w16943:bool)
            n10272 = local read "Ch2_Cst_fix_do"() -> (w16942:bool)
            n10273 = Exclusive Or(1:w16943, 2:w16942) -> (0:w16946:bool)
            n10274 = feedback #398() -> (w16944:bool)  [unwired: 1 in]
            n10275 = case shown="True" w16946 {
              tunnel: [TRUE FALSE] -> w16945
              tunnel: w16944 -> [_ w16970]
              tunnel: [FALSE w16967] -> w16941
              frame #0 {
              }
              frame #1 {
                n10276 = call "Elapsed Time187"("Reset"=w16970) -> ("Elapsed Time (s)"=w16969:dbl)  [unwired: 11 in, 7 out]
                n10277 = Greater?(x=w16969, y=60.0) -> (0:w16967:bool)
              }
            }
            n10278 = local write "chamber 2top piston failed"(w16941) -> ()
          }
        }
        n10279 = case shown="False" w16921 {
          frame #0 {
            w16993 = TRUE
            n10280 = local write "Ch2_Bg_bv_fail"(w16993) -> ()
            n10281 = local write "Ch2_Mp_fail"(w16993) -> ()
            n10282 = local write "Ch2_Tp_bv_fail"(w16993) -> ()
            n10283 = local write "Ch2_Ch_vbv_fail"(w16993) -> ()
            n10284 = local write "Ch2_Ch_atm_fail"(w16993) -> ()
            n10285 = local write "ch2_atm_fail_top"(w16993) -> ()
            n10286 = local write "Ch2_Pl_atm_fail"(w16993) -> ()
            n10287 = local write "Ch2_Ch_cc_fail"(w16993) -> ()
            n10288 = local write "ch2_bg_bv_fail_top"(w16993) -> ()
            n10289 = local write "ch2_cc_fail_top"(w16993) -> ()
            n10290 = local write "Ch2_Pl_vbv_fail"(w16993) -> ()